vi "rydberg_trigger_snap.vi"() -> ()   [LabVIEW 2013] (continued)
  # "Applies to 1D arbitrary fit."
  # "Number of columns and rows at the\ncorners to find uncertainties/noise."
  # "Number of pixels in smoothing\nfor plotting residuals."
  # "Isotope"
  # "Avg. Temp (uK)"
  # "Drop Time (ms)"
  # "<-------- toward source <----------"
  # "<-------- toward source <----------"
  # "gravity\n  |\n  |\n  |\n  V"
  # "MAXIMUM COUNTS FOR PIXELFLY \nSINGLE SHOT: 4096"
  # "gravity\n  |\n  |\n  |\n  V"
  # "<-------- toward source <----------"
  # "2D Fitting"
  # "1D Fitting"
  # "x                  y"
  # "Camera Indicators\nto Ignore"
  # "Status flags"
  # "Buffer errors"
  # "Memory usage"
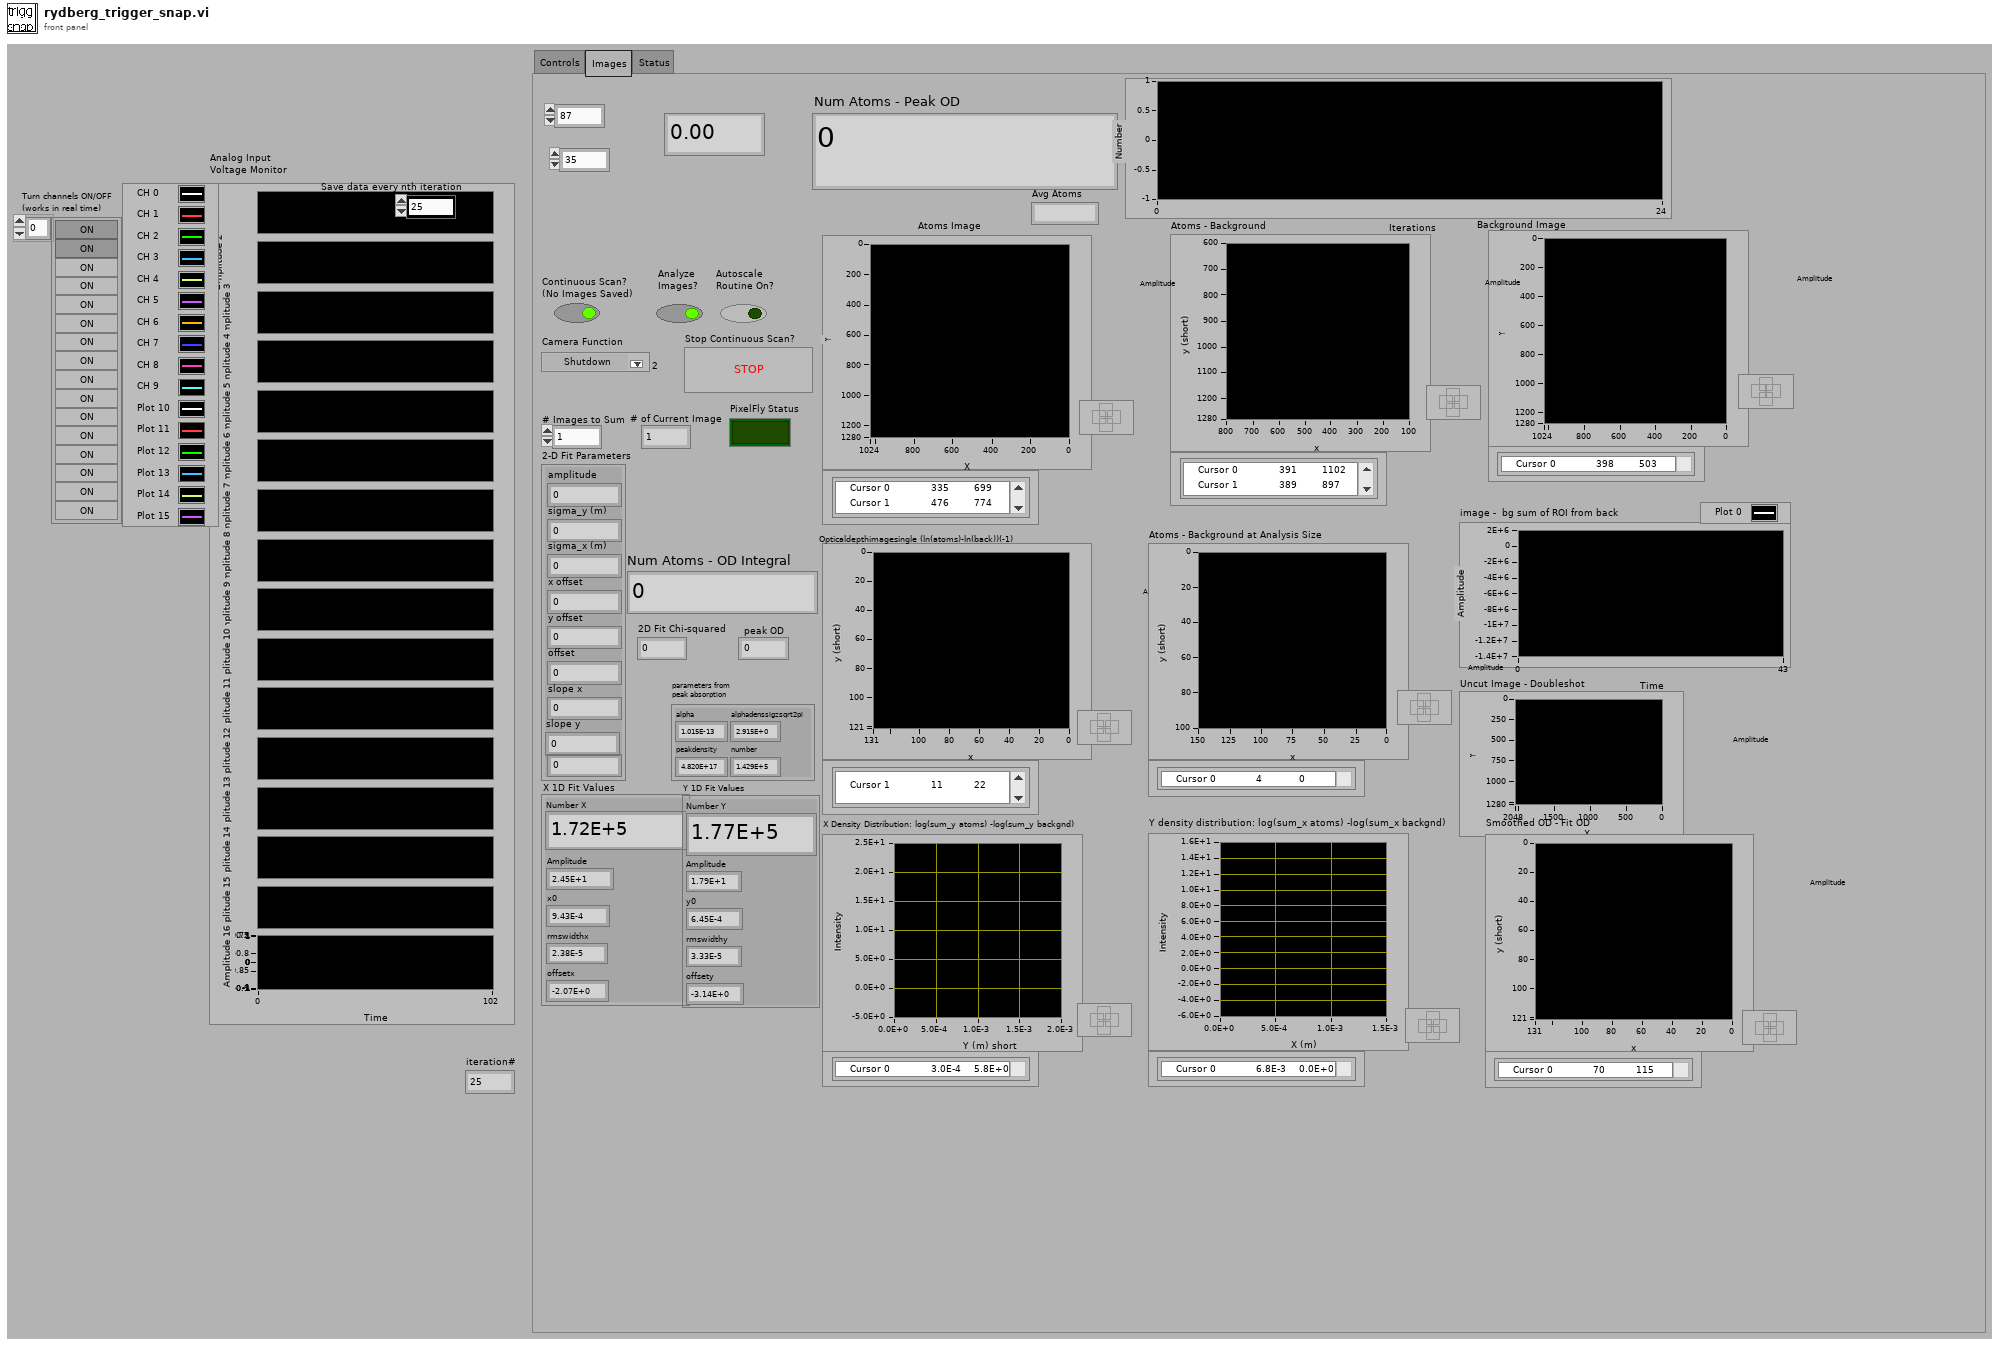
[diagram p1: front panel]
types:
  T1 = cluster{"data[0]":dbl, "data[1]":dbl, "data[2]":dbl, "data[3]":dbl, "data[4]":dbl, "data[5]":dbl, "data[6]":dbl, "data[7]":dbl, "data[8]":dbl, "data[9]":dbl, "data[10]":dbl, "data[11]":dbl, "data[12]":dbl, "data[13]":dbl, "data[14]":dbl, "data[15]":dbl}
  T2 = cluster{"Col Start":i32, "Col Stop":i32, "Row Start":i32, "Row stop":i32}
  T3 = cluster{"alpha":dbl, "peakdensity":dbl, "alphadenssigzsqrt2pi":sgl, "number":dbl}
  T4 = cluster{"Amplitude":dbl, "y0":dbl, "rmswidthy":dbl, "offsety":dbl, "Number Y":dbl}
  T5 = cluster{"Amplitude":dbl, "x0":dbl, "rmswidthx":dbl, "offsetx":dbl, "Number X":dbl}
  T6 = cluster{"amplitude":dbl, "sigma_y (m)":dbl, "sigma_x (m)":dbl, "x offset":dbl, "y offset":dbl, "offset":dbl, "slope x":dbl, "slope y":dbl, dbl}
  T7 = cluster{"Type":u32, "Number":u32, "Initialized":bool, "Running":bool, "Lost head":bool, "CCD X size":u32, "CCD Y size":u32, "Mode":u32, "Exposure time":u32, "Exposure level":u32, "Horizontal bin":u32, "Vertical bin":u32, "Reg W":bool, "Gain":u32, "Pixel depth":i32, "Bit Shift":u32, "Offset":u32, "Last exposure":u32, "Double ":bool, "Light meter":bool, "Color":bool, "Open count":u32, "Active buffer":bool, "Next Buffer":bool}
  T8 = cluster{"Write":bool, "Write done":bool, "Queued":bool, "Cancelled":bool, "Select":bool, "Select done":bool, "Burst":bool, "Size":bool, "Event":bool, "Timeout":bool, "Open":i32, "Map":i32, "Exposure":i32[], "Offset":i32[], "Size":i32[], "Transfer":i32[], "Total Size":i32}
  T9 = cluster{"amplitudey":dbl, "temperaturey":dbl, "alphay":dbl, "offsety":dbl, "numbery":dbl, "peakdensityy":dbl, "centery":dbl}
  T10 = cluster{"amplitudex":dbl, "temperaturex":dbl, "alphax":dbl, "offsetx":dbl, "numberx":dbl, "peakdensityx":dbl, "centerx":dbl}
  T11 = cluster{"ccdxsize":i32, "ccdy":i32, "pictx":i32, "picty":i32, "bitspixel":i32}
  T12 = cluster{"Type":u32, "Number":u32, "Initialized":bool, "Running":bool, "Lost head":bool, "CCD X size":u32, "CCD Y size":u32, "Mode":u32, "Exposure time":u32, "Exposure level":u32, "Horizontal bin":u32, "Vertical bin":u32, "Reg W":bool, "Gain":u32, "Pixel depth":i32, "Bit Shift":u32, "Offset":u32, "Last exposure":u32, "Double":bool, "Light meter":bool, "Color":bool, "Open count":u32, "Active buffer":bool, "Next Buffer":bool}
  T13 = cluster{"Sample Interleave":dbl, "Pixel Size (m)":dbl, i32, "Cut Borders":dbl, "Number for Scale":dbl, "Limit":dbl, "Number of Pixels to Smooth":dbl}
  T14 = cluster{"abscrosssection":dbl, "peakdensity":dbl, "twosizeoneoverezabsxsecdens":dbl, "number":dbl}
  T15 = cluster{"Amplitude":dbl, "x0":dbl, "rmswidthx":dbl, "offsetx":dbl, "numberx":dbl}
  T16 = cluster{"Amplitude":dbl, "y0":dbl, "rmswidthy":dbl, "offsety":dbl, "numbery":dbl}
  T17 = cluster{"amplitude":dbl, "sigma_y (m)":dbl, "sigma_x (m)":dbl, "row offset (pixel #)":dbl, "col offset (pixel #)":dbl, "offset":dbl, "slope x":dbl, "slope y":dbl, dbl}
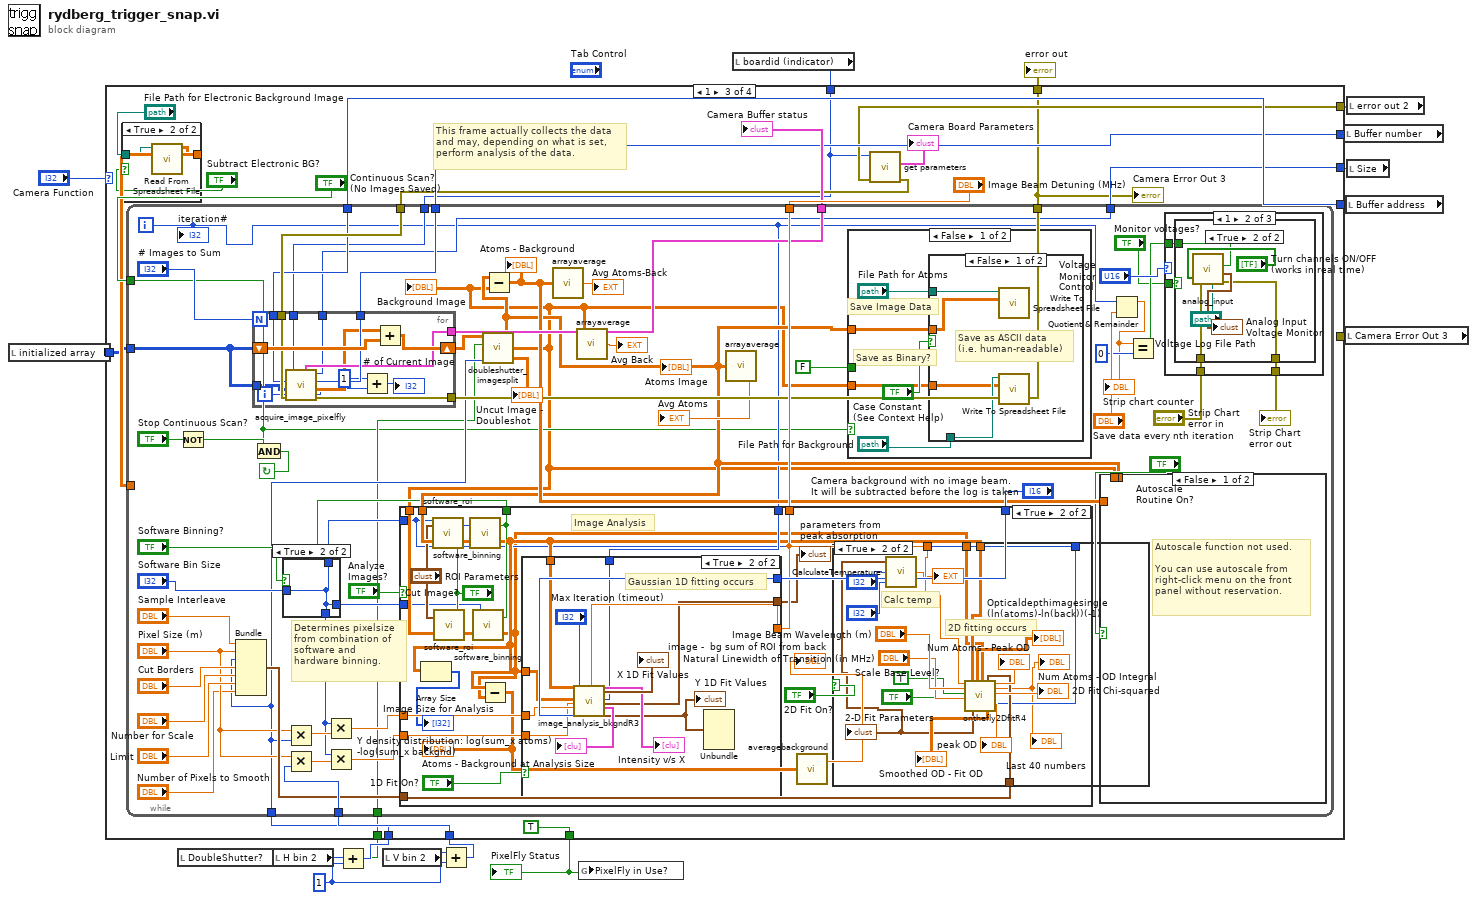
[diagram p0: block diagram]
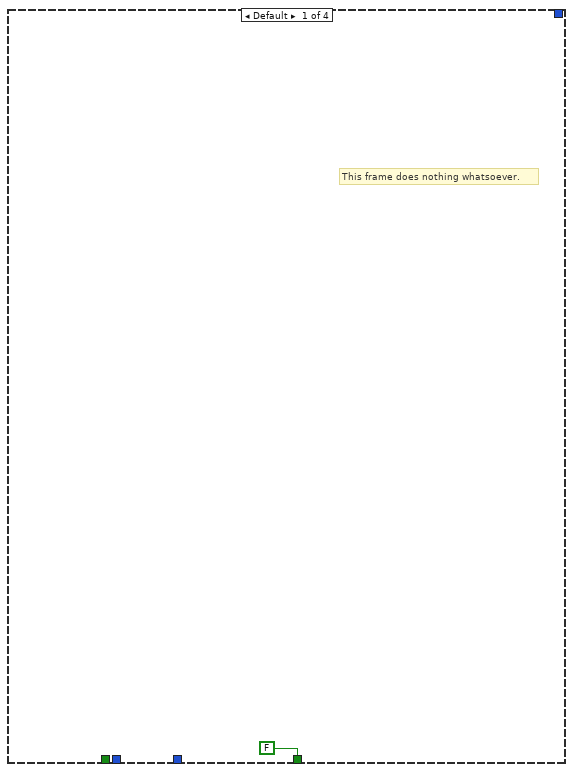
[diagram p2: hidden frame]
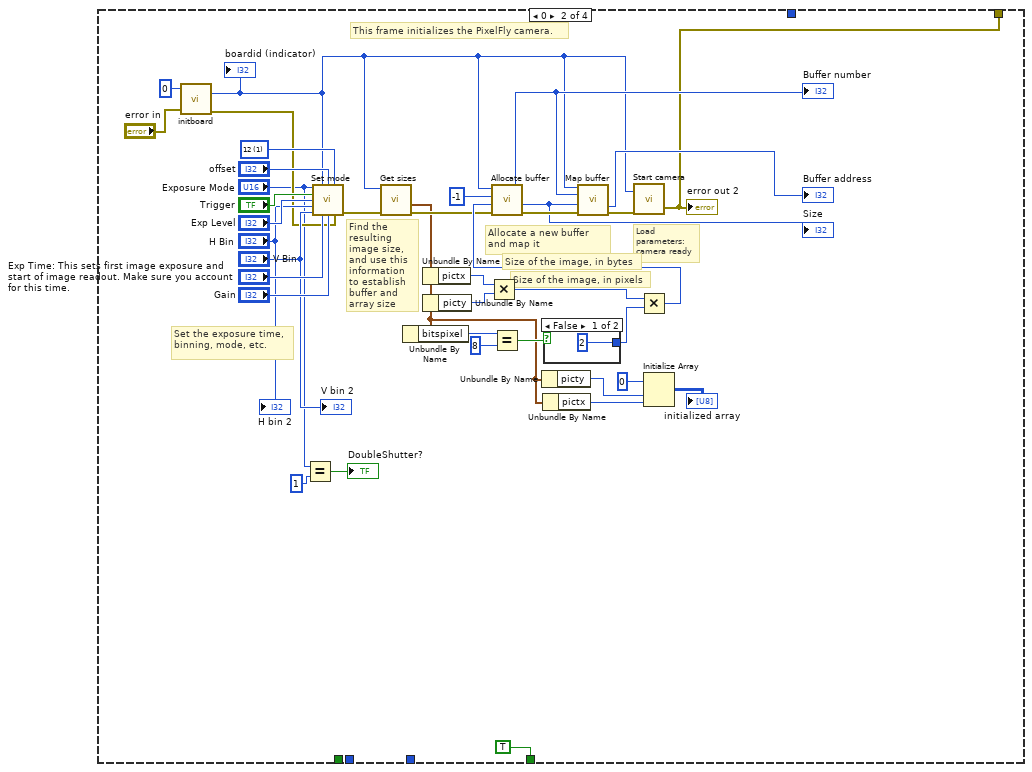
[diagram p3: hidden frame]
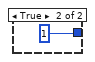
[diagram p4: hidden frame]
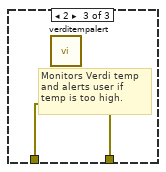
[diagram p8: hidden frame]
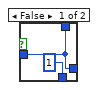
[diagram p9: hidden frame]
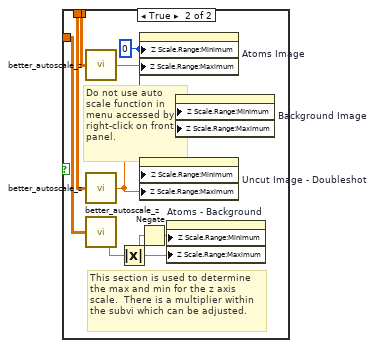
[diagram p10: hidden frame]
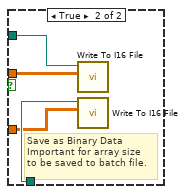
[diagram p11: hidden frame]
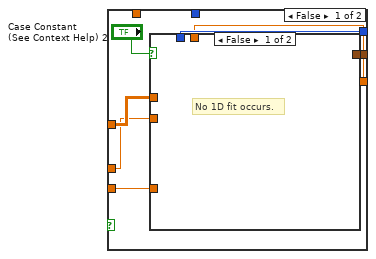
[diagram p15: hidden frame]
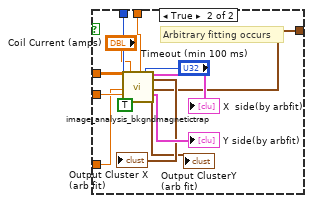
[diagram p16: hidden frame]
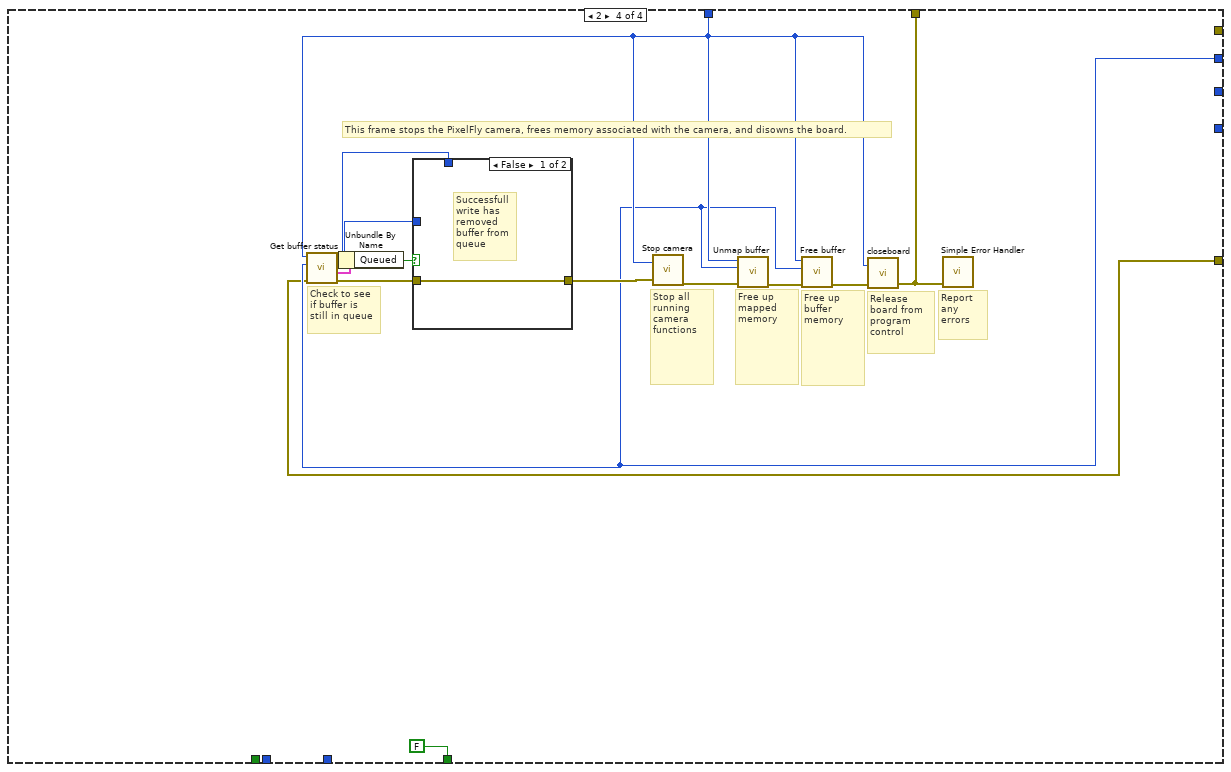
[diagram p17: hidden frame]
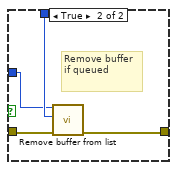
[diagram p18: hidden frame]
diagram:
  w5 = 1
  n1 = local read "initialized array"() -> (w3:u8[][])
  n2 = local read "DoubleShutter?"() -> (w2:bool)
  n3 = local read "H bin 2"() -> (w8:i32)
  n4 = Add(x=w8, y=w5) -> (x+y=w7:i32)
  n5 = local read "V bin 2"() -> (w6:i32)
  n6 = Add(x=w6, y=w5) -> (x+y=w4:i32)
  n7 = local read "boardid (indicator)"() -> (w9:i32)
  n8 = local read "Buffer number"() -> (w11:i32)
  n9 = local read "Camera Error Out 3"() -> (w14:errorcluster)
  n10 = local read "Buffer address"() -> (w13:i32)
  n11 = local read "error out 2"() -> (w15:errorcluster)
  n12 = local read "Size"() -> (w12:i32)
  n13 = case shown="1" "Camera Function" {
    tunnel: w15 -> [_ _ w67 _]
    tunnel: w14 -> [_ _ _ w261]
    tunnel: w13 -> [_ _ w74 _]
    tunnel: w12 -> [_ _ w73 _]
    tunnel: w11 -> [_ _ w71 w262]
    tunnel: w7 -> [_ _ w69 _]
    tunnel: w4 -> [_ _ w70 _]
    tunnel: [_ w26 w65 w264] -> w10
    tunnel: w9 -> [_ _ w64 w263]
    tunnel: w3 -> [_ _ w61 _]
    tunnel: w2 -> [_ _ w60 _]
    tunnel: [FALSE TRUE TRUE FALSE] -> w1
    frame Default {
      # "This frame does nothing whatsoever."
    }
    frame 0 {
      w37 = 1 items=["8", "12"] ("bits/pixel")
      # "This frame initializes the PixelFly camera."
      # "Load parameters: camera ready"
      # "Allocate a new buffer and map it"
      # "Set the exposure time, binning, mode, etc."
      # "Find the resulting image size, and use this information to establish buffer and array size"
      # "Size of the image, in pixels"
      # "Size of the image, in bytes"
      n14 = call "initboard.vi"("boardid in"=0, "error in (no error)"="error in") -> ("boardid"=w23:i32, "error out"=w22:errorcluster)  [unwired: 2 in, 1 out]
      "boardid (indicator)" <- w23
      n15 = Equal?(x="Exposure Mode", y=1) -> (x = y?=→"DoubleShutter?":bool)
      n16 = call "Set mode.vi"("Exposure mode"="Exposure Mode", "Handle in"=w23, "offset"="offset", "bits/pixel"=w37, "trigger"="Trigger", "exp level"="Exp Level", "H bin"="H Bin", "V bin"="V Bin", "exp time"="Exp Time: This sets first image exposure and start of image readout. Make sure you account for this time.", "gain"="Gain", "error in (no error)"=w22) -> ("error out"=w50:errorcluster)  [unwired: 4 in]
      n17 = call "Get sizes.vi"("Handle in"=w23, "error in (no error)"=w50) -> ("Picture parameters"=w36:T11, "error out"=w41:errorcluster)  [unwired: 1 in, 2 out]
      n18 = Unbundle By Name(w36) -> ("bitspixel"=w47:i32)
      n19 = Unbundle By Name(w36) -> ("pictx"=w49:i32)
      n20 = Unbundle By Name(w36) -> ("picty"=w48:i32)
      n21 = Multiply(x=w49, y=w48) -> (x*y=w44:i32)
      n22 = Equal?(x=w47, y=8) -> (x = y?=w45:bool)
      n23 = Unbundle By Name(w36) -> ("picty"=w29:i32)
      n24 = Unbundle By Name(w36) -> ("pictx"=w28:i32)
      n25 = case shown="False" w45 {
        tunnel: [2 1] -> w43
        frame False {
        }
        frame True {
        }
      }
      n26 = Multiply(x=w44, y=w43) -> (x*y=w42:i32)
      n27 = call "Allocate buffer.vi"("error in (no error)"=w41, "Size request"=w42, "Buffer request"=-1, "Handle in"=w23) -> ("error out"=w39:errorcluster, "Size"=w34:i32, "Buffer number"=w33:i32)  [unwired: 1 out]
      "Size" <- w34
      "Buffer number" <- w33
      n28 = call "Map buffer.vi"("Handle in"=w23, "Buffer in"=w33, "size"=w34, "error in (no error)"=w39) -> ("Buffer address"=→"Buffer address":i32, "error out"=w35:errorcluster)  [unwired: 8 in, 2 out]
      n29 = call "Start camera.vi"("Handle in"=w23, "error in (no error)"=w35) -> ("error out"=w26:errorcluster)  [unwired: 2 out]
      "error out 2" <- w26
      n30 = Initialize Array(u8 0 ("16 bit integers"), w29, w28) -> (→"initialized array":u8[][])
      "H bin 2" <- "H Bin"
      "V bin 2" <- "V Bin"
    }
    frame 1 {
      # "This frame actually collects the data\nand may, depending on what is set,\nperform analysis of the data."
      n31 = case shown="True" "Subtract Electronic BG?" {
        tunnel: "File Path for Electronic Background Image" -> [_ w78]
        tunnel: [_ w77] -> w62
        frame False {
        }
        frame True {
          n32 = call-poly <vilib>:"Read From Spreadsheet File.vi"("file path (dialog if empty)"=w78) -> ("all rows"=w77:dbl[][])  [unwired: 6 in, 4 out]
        }
      }
      n33 = call "get parameters.vi"("error in (no error)"=w67, "Handle in"=w64) -> ("error out"=w68:errorcluster, "Board Parameters"=→"Camera Board Parameters":T12)  [unwired: 2 in, 2 out]
      n34 = while {
        tunnel: "Image Beam Detuning (MHz)" -> [w132]
        tunnel: w68 -> [w131]
        tunnel: "Continuous Scan?\n(No Images Saved)" -> [w80]
        tunnel: [w128] -> w65
        tunnel: w74 -> [w126]
        tunnel: w64 -> [w125]
        tunnel: w73 -> [w90]
        tunnel: w71 -> [w124]
        tunnel: [w123] -> w72
        tunnel: w70 -> [w122]
        tunnel: w69 -> [w85]
        tunnel: w62 -> [_]
        tunnel: w61 -> [w107]
        tunnel: w60 -> [w81]
        i -> [w86]
        stop <- w130 continue-if-true
        # "Determines pixelsize\nfrom combination of\nsoftware and\nhardware binning."
        n35 = Not(x="Stop Continuous Scan?") -> (.not. x?=w127:bool)
        n36 = Bundle("Sample Interleave"="Sample Interleave", "Pixel Size (m)"="Pixel Size (m)", w85, "Cut Borders"="Cut Borders", "Number for Scale"="Number for Scale", "Limit"="Limit", "Number of Pixels to Smooth"="Number of Pixels to Smooth") -> (w110:T13)  [unwired: 1 in]
        n37 = for {
          N: "# Images to Sum" -> [_]
          tunnel: w131 -> [w168]
          shift-right: [w171] -> w114
          shift-left: w107 -> [w170]
          tunnel: [w169] -> w128
          tunnel: w126 -> [w167]
          tunnel: w125 -> [w166]
          tunnel: w124 -> [w165]
          tunnel: [w164] -> w123
          tunnel: w90 -> [w162]
          tunnel: w107 -> [w158]
          i -> [w161]
          n38 = call "acquire_image_pixelfly.vi"("boardid"=w166, "Buffer address"=w167, "Array input"=w158, "error in"=w168, "Size"=w162, "Buffer number"=w165) -> ("Buffer status"=w164:T8, "image array"=w163:dbl[][], "error out"=w169:errorcluster)
          n39 = Add(x=1, y=w161) -> (x+y=→"# of Current Image":i32)
          n40 = Add(x=w163, y=w170) -> (x+y=w171:dbl[][])
        }
        n41 = And(x=w127, y=w80) -> (x .and. y?=w130:bool)
        n42 = case shown="True" "Software Binning?" {
          tunnel: [w147 w148] -> w98
          tunnel: "Software Bin Size" -> [w147 w148]
          tunnel: [w147 w148] -> w96
          tunnel: [1 w148] -> w95
          frame False {
          }
          frame True {
          }
        }
        n43 = Multiply(x="Pixel Size (m)", y=w85) -> (x*y=w113:dbl)
        n44 = Multiply(x="Pixel Size (m)", y=w122) -> (x*y=w112:dbl)
        n45 = Multiply(x=w95, y=w113) -> (x*y=w109:dbl)
        n46 = Multiply(x=w95, y=w112) -> (x*y=w111:dbl)
        n47 = call "doubleshutter_imagesplit.vi"("image array"=w114, "DoubleShutter?"=w81, "x bin"=w85) -> ("lower half - atoms"=w99:dbl[][], "upper half - background"=w79:dbl[][], "Uncut Image"=→"Uncut Image - Doubleshot":dbl[][])  [unwired: 2 in]
        "Atoms Image" <- w99
        "Background Image" <- w79
        n48 = case shown="True" "Analyze \nImages?" {
          tunnel: w109 -> [_ w197]
          tunnel: w111 -> [_ w196]
          tunnel: "Camera background with no image beam.\nIt will be subtracted before the log is taken" -> [_ w207]
          tunnel: w132 -> [_ w205]
          tunnel: w86 -> [_ w206]
          tunnel: w110 -> [_ w204]
          tunnel: w99 -> [_ w201]
          tunnel: w79 -> [_ w198]
          tunnel: w96 -> [_ w189]
          tunnel: "Software Binning?" -> [_ w192]
          tunnel: w98 -> [_ w191]
          frame False {
            # "Perform No Analysis"
            # "No analysis done."
          }
          frame True {
            # "Image Analysis"
            n49 = call "software_roi.vi"("Cut image?"="Cut Image?", "Input Array"=w201, "ROI Controls"="ROI Parameters") -> ("output array"=w194:sgl[][])
            n50 = call "software_roi.vi"("Cut image?"="Cut Image?", "Input Array"=w198, "ROI Controls"="ROI Parameters") -> ("output array"=w193:sgl[][])
            n51 = call "software_binning.vi"("Bin image?"=w192, "Input Array"=w194, "bin size"=w189) -> ("Binned Array"=w190:dbl[][])
            n52 = Array Size(array=w190) -> (size(s)=→"Image Size for Analysis":i32[])
            n53 = call "software_binning.vi"("Bin image?"=w192, "Input Array"=w193, "bin size"=w191) -> ("Binned Array"=w188:dbl[][])
            n54 = Subtract(x=w190, y=w188) -> (x-y=w187:dbl[][])
            "Atoms - Background at Analysis Size" <- w187
            n55 = case shown="True" "1D Fit On?" {
              tunnel: w188 -> [w231 w249]
              tunnel: w207 -> [w233 w254]
              tunnel: w205 -> [w232 w258]
              tunnel: w190 -> [_ w250]
              tunnel: w206 -> [_ w253]
              tunnel: w197 -> [w229 w252]
              tunnel: w196 -> [w228 w251]
              tunnel: [w227 w247] -> w185
              frame False {
                n56 = case shown="False" "Case Constant\n(See Context Help) 2" {
                  tunnel: w229 -> [_ w245]
                  tunnel: w228 -> [_ w244]
                  tunnel: w233 -> [_ w243]
                  tunnel: w232 -> [_ w241]
                  tunnel: w231 -> [_ w236]
                  tunnel: [_ w234] -> w227
                  frame False {
                    # "No 1D fit occurs."
                  }
                  frame True {
                    # "Arbitrary fitting occurs"
                    n57 = call "image_analysis_bkgndmagnetictrap.vi"("2D Array In"=w236, "Delta_x (m)"=w244, "Delta_y (m)"=w245, "camera background with no image beam\nIt will be subtracted before the log is taken"=w243, "coilcurrent"="Coil Current (amps)", "take new\nnew image"=TRUE ("take new\nnew image"), "Image beam \nDetuning (MHz)"=w241, "timeout(min 100ms)"="Timeout (min 100 ms)") -> ("X  side"=→"X  side(by arbfit)":cluster{cluster{dbl, dbl}[]}[], "Output Cluster X"=→"Output Cluster X\n(arb fit)":T10, "parameters from\n peak absorption"=w234:T14, "Y side"=→"Y side(by arbfit)":cluster{cluster{dbl, dbl}[]}[], "Output ClusterY"=→"Output ClusterY\n(arb fit)":T9)  [unwired: 5 in, 2 out]
                  }
                }
              }
              frame True {
                # "Gaussian 1D fitting occurs"
                n58 = call "image_analysis_bkgndR3.vi"("Atoms array in"=w250, "BG array in"=w249, "Delta_x (m)"=w251, "Delta_y (m)"=w252, "camera background with no image beam\nIt will be subtracted before the log is taken"=w254, "max iteration"="Max Iteration (timeout)", "Image beam \nDetuning (MHz)"=w258, "Iteration #"=w253) -> ("Intensity v/s X 2"=→"Intensity v/s X":cluster{dbl[], dbl[]}[], "x fit values"=→"X 1D Fit Values":T15, "parameters from \npeak absorption"=w247:T3, "Intensity v/s X"=→"Y density distribution: log(sum_x atoms) -log(sum_x backgnd)":cluster{dbl[], dbl[]}[], "y fit values"=w248:T16)  [unwired: 13 in, 2 out]
                "Y 1D Fit Values" <- w248
                n59 = Unbundle(w248) -> ()  [unwired: 5 out]
              }
            }
            "parameters from \npeak absorption" <- w185
            n60 = call "averagebackground.vi"("Input Array"=w187) -> ("sum of Gaussian"=→"image -  bg sum of ROI from back":dbl)  [unwired: 1 out]
            n61 = case shown="True" "2D Fit On?" {
              tunnel: w190 -> [_ w216]
              tunnel: w205 -> [_ w212]
              tunnel: w204 -> [_ w221]
              tunnel: w188 -> [_ w215]
              tunnel: w189 -> [_ w214]
              frame False {
                # "No 2D fitting occurs"
              }
              frame True {
                # "Calc temp"
                # "2D fitting occurs"
                n62 = call "onthefly2DfitR4.vi"("Detuning in MHz"=w212, "Wavelength (m)"="Image Beam Wavelength (m)", "pass image method"=TRUE, "Natural Linewidth of Transition\n(ion fwhm in MHz)"="Natural Linewidth of Transition (in MHz)", "Scale Base Level?"="Scale Base Level?", "Atoms"=w216, "Background"=w215, "Specifics of Fitting Routines"=w221, "Software bin size"=w214) -> ("2-D Gaussian Fit Parameters"=w208:T17, "opticaldepthimagesingle\n(ln(atoms)-ln(back))(-1)"=→"Opticaldepthimagesingle (ln(atoms)-ln(back))(-1)":dbl[][], "peak OD"=→"peak OD":dbl, "smoothed OD-fit OD"=→"Smoothed OD - Fit OD":dbl[][], "# atoms from peakOD"=→"Num Atoms - Peak OD":dbl, "# atoms from \nODintegral"=→"Num Atoms - OD Integral" →"Last 40 numbers":dbl, "Chi-squared"=→"2D Fit Chi-squared":dbl)  [unwired: 2 in, 2 out]
                "2-D Fit Parameters" <- w208
                n63 = call "CalculateTemperature.vi"("Droptime (ms)"="?", "Isotope"="?", "2-D Fit Parameters"=w208) -> ("Avg. Temp"=→"?":ext)
              }
            }
          }
        }
        n64 = Subtract(x=w99, y=w79) -> (x-y=w108:dbl[][])
        "Atoms - Background" <- w108
        n65 = call "arrayaverage.vi"("Array int 32"=w108) -> ("Average"=→"Avg Atoms-Back":ext)
        n66 = call "arrayaverage.vi"("Array int 32"=w79) -> ("Average"=→"Avg Back":ext)
        n67 = call "arrayaverage.vi"("Array int 32"=w99) -> ("Average"=→"Avg Atoms":ext)
        n68 = case shown="False" w80 {
          tunnel: w99 -> [w173 _]
          tunnel: w79 -> [w172 _]
          tunnel: FALSE -> [_ _]
          frame False {
            # "Save as Binary?"
            # "Save Image Data"
            n69 = case shown="False" "Case Constant\n(See Context Help)" {
              tunnel: "File Path for Atoms" -> [w180 w184]
              tunnel: "File Path for Background" -> [w179 w183]
              tunnel: w173 -> [w178 w181]
              tunnel: w172 -> [w177 w182]
              frame False {
                # "Save as ASCII data\n(i.e. human-readable)"
                n70 = call-poly <vilib>:"Write To Spreadsheet File.vi"("2D data"=w178, "file path (dialog if empty)"=w180) -> ()  [unwired: 6 in, 1 out]
                n71 = call-poly <vilib>:"Write To Spreadsheet File.vi"("2D data"=w177, "file path (dialog if empty)"=w179) -> ()  [unwired: 6 in, 1 out]
              }
              frame True {
                # "Save as Binary Data\nImportant for array size\nto be saved to batch file."
                n72 = call <vilib>:"Write To I16 File.vi"("2D array"=w181, "file path (dialog if empty)"=w184) -> ()  [unwired: 5 in, 1 out]
                n73 = call <vilib>:"Write To I16 File.vi"("2D array"=w182, "file path (dialog if empty)"=w183) -> ()  [unwired: 5 in, 1 out]
              }
            }
          }
          frame True {
            # "Don't Save Data\nWhen Continous"
          }
        }
        n74 = case shown="False" "Autoscale\nRoutine On?" {
          tunnel: w99 -> [_ w157]
          tunnel: w79 -> [_ w155]
          tunnel: w108 -> [_ w153]
          frame False {
            # "Autoscale function not used.\n\nYou can use autoscale from\nright-click menu on the front\npanel without reservation."
          }
          frame True {
            w152 = 0
            # "Do not use auto\nscale function in\nmenu accessed by\nright-click on front\npanel."
            # "This section is used to determine\nthe max and min for the z axis\nscale.  There is a multiplier within\nthe subvi which can be adjusted."
            n75 = call "better_autoscale_z.vi"("Input Array"=w157) -> ("autoscale max"=w156:dbl)
            n76 = call "better_autoscale_z.vi"("Input Array"=w155) -> ("autoscale max"=w154:dbl)
            n77 = call "better_autoscale_z.vi"("Input Array"=w153) -> ("autoscale max"=w151:dbl)
            n78 = Absolute Value(x=w151) -> (abs(x)=w149:dbl)
            n79 = Negate(x=w149) -> (-x=w150:dbl)
            n80 = property on="Atoms Image" class="IntGraph (strict)"("Z Scale.Range:Minimum"=w152, "Z Scale.Range:Maximum"=w156) -> ()  [unwired: 2 in, 2 out]
            n81 = property on="Uncut Image - Doubleshot" class="IntGraph (strict)"("Z Scale.Range:Minimum"=w152, "Z Scale.Range:Maximum"=w154) -> ()  [unwired: 2 in, 2 out]
            n82 = property on="Atoms - Background" class="IntGraph (strict)"("Z Scale.Range:Minimum"=w150, "Z Scale.Range:Maximum"=w149) -> ()  [unwired: 2 in, 2 out]
            n83 = property on="Background Image" class="IntGraph (strict)"("Z Scale.Range:Minimum"=w152, "Z Scale.Range:Maximum"=w154) -> ()  [unwired: 2 in, 2 out]
          }
        }
        n84 = Quotient & Remainder(x=w86, y="Save data every nth iteration") -> (x-y*floor(x/y)=w87:dbl)  [unwired: 1 out]
        "Strip chart counter" <- w87
        n85 = Equal?(x=w87, y=0) -> (x = y?=w84:bool)
        n86 = case shown="1" "Voltage\nMonitor\nControl" {
          tunnel: "Strip Chart\nerror in" -> [w133 w137 w145]
          tunnel: [w133 w136 w145] -> w91
          tunnel: "Monitor voltages?" -> [_ w135 _]
          tunnel: w84 -> [_ w134 _]
          frame 0, Default {
          }
          frame 1 {
            n87 = case shown="True" w135 {
              tunnel: w137 -> [w138 w143]
              tunnel: [w138 w142] -> w136
              tunnel: w134 -> [_ w139]
              frame False {
              }
              frame True {
                n88 = call "analog_input.vi"("save values?"=w139, "Voltage Log File Path"="Voltage Log File Path", 5:"Turn channels ON/OFF\n(works in real time)", "error in"=w143) -> ("error out"=w142:errorcluster, "Data display"=→"Analog Input \nVoltage Monitor":T1)  [unwired: 1 out]
              }
            }
          }
          frame 2 {
            # "Monitors Verdi temp\nand alerts user if\ntemp is too high."
            n89 = call "verditempalert.vi"() -> ()  [unwired: 1 in]
          }
        }
        "Strip Chart\nerror out" <- w91
        "iteration#" <- w86
      }
      "Camera Error Out 3" <- w65
      "Camera Buffer status" <- w72
    }
    frame 2 {
      # "This frame stops the PixelFly camera, frees memory associated with the camera, and disowns the board."
      # "Check to see if buffer is still in queue"
      # "Report any errors"
      # "Release board from program control"
      # "Free up buffer memory"
      # "Free up mapped memory"
      # "Stop all running camera functions"
      n90 = call "Get buffer status.vi"("error in (no error)"=w261, "Buffer request"=w262, "Handle in"=w263) -> ("error out"=w269:errorcluster, "Buffer status"=w270:T8, "Buffer number"=w266:i32, "Handle out"=w265:i32)  [unwired: 1 in]
      n91 = Unbundle By Name(w270) -> ("Queued"=w268:bool)
      n92 = case shown="False" w268 {
        tunnel: w269 -> [w274 w278]
        tunnel: [w274 w277] -> w267
        tunnel: w266 -> [_ w276]
        tunnel: w265 -> [_ w275]
        frame False {
          # "Successfull write has removed buffer from queue"
        }
        frame True {
          # "Remove buffer if queued"
          n93 = call "Remove buffer from list.vi"("error in (no error)"=w278, "Buffer in"=w276, "Handle in"=w275) -> ("error out"=w277:errorcluster)  [unwired: 2 in, 2 out]
        }
      }
      n94 = call "Stop camera.vi"("Handle in"=w263, "error in (no error)"=w267) -> ("error out"=w272:errorcluster)  [unwired: 2 out]
      n95 = call "Unmap buffer.vi"("error in (no error)"=w272, "Buffer in"=w262, "Handle in"=w263) -> ("error out"=w273:errorcluster)  [unwired: 2 in, 2 out]
      n96 = call "Free buffer.vi"("error in (no error)"=w273, "Buffer in"=w262, "Handle in"=w263) -> ("error out"=w271:errorcluster)  [unwired: 2 in, 2 out]
      n97 = call "closeboard.vi"("Handle in"=w263, "error in (no error)"=w271) -> ("error out"=w264:errorcluster)  [unwired: 2 out]
      n98 = call <vilib>:"Simple Error Handler.vi"("error in (no error)"=w264) -> ()  [unwired: 4 in, 5 out]
    }
  }
  "error out" <- w10
  "PixelFly Status" <- w1
  n99 = global write "check_pixelfly_status.vi" "PixelFly in Use?"(w1) -> ()
